vi "pp2_videoQueueMake.vi"(8 "error in":errorcluster, 11 "Camera":T3="cam0") -> (0 "error out":errorcluster, 1 "Image reference":T4, 2 "Session Out":T3, 3 "queue out":refnum<queue>)   [LabVIEW 2013]
uses:
  <vilib>/userdefined/High Color/IMAQdx.ctl
  <vilib>/vision/Image Controls.llb/IMAQ Image.ctl
  pp2_CTL_DaqConfig.ctl
  <vilib>/sound2/lvsound2.llb/Sound Output Task ID.ctl
  <vilib>/vision/driver/NI_Vision_Acquisition_Software.lvlib
panel:
  in  "Daq config 2":T1={"SW1 DI"="Dev1/port2/line0", "Code/Tone DO"="Dev1/port0:1", "Sound AO"="Dev2/ao0", "Shock intesity AO"="Dev1/ao1", "SW2 DI"="Dev1/port2/line1", "AO <=> Sound card"=FALSE, "sound card task"=0, "Variable shock"=FALSE, "Full code <=> Tone"=FALSE, "Webcam"="cam0", "Webcam on"=FALSE, "sound sample rate"=8000, "sound card\ndevice ID"=0} {"sound sample rate" min=8000; "sound card task" format="%.0x"}
  in  "Daq config":T1={"SW1 DI"="Dev1/port2/line0", "Code/Tone DO"="Dev1/port0:1", "Sound AO"="Dev2/ao0", "Shock intesity AO"="Dev1/ao1", "SW2 DI"="Dev1/port2/line1", "AO <=> Sound card"=FALSE, "sound card task"=0, "Variable shock"=FALSE, "Full code <=> Tone"=FALSE, "Webcam"="cam0", "Webcam on"=FALSE, "sound sample rate"=8000, "sound card\ndevice ID"=0} {"sound sample rate" min=8000; "sound card task" format="%.0x"}
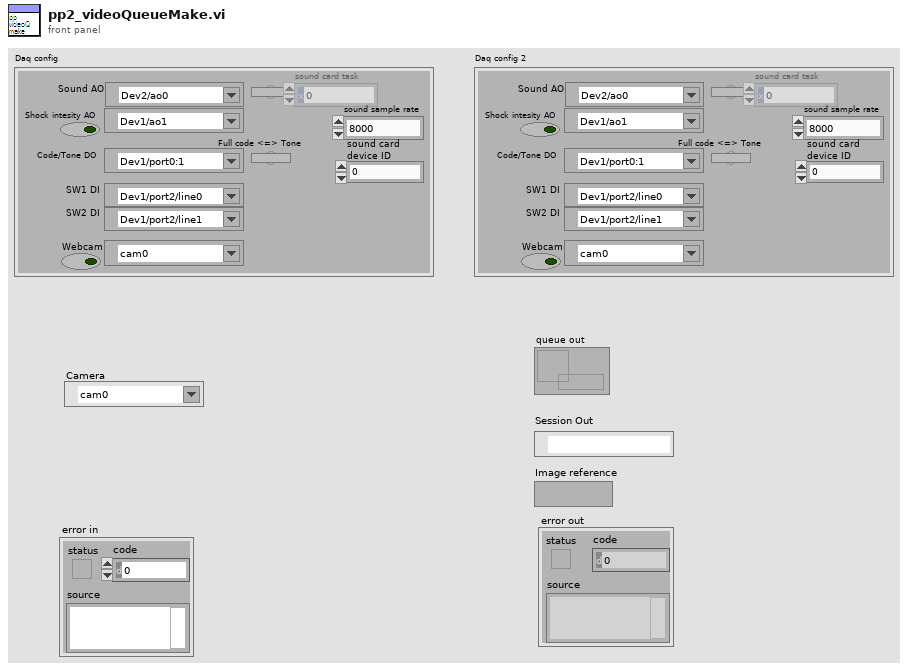
[diagram p1: front panel]
types:
  T1 = typedef "pp2_CTL_DaqConfig.ctl" = cluster{"SW1 DI":tag, "Code/Tone DO":tag, "Sound AO":tag, "Shock intesity AO":tag, "SW2 DI":tag, "AO <=> Sound card":bool, "sound card task":T2, "Variable shock":bool, "Full code <=> Tone":bool, "Webcam":T3, "Webcam on":bool, "sound sample rate":i32, "sound card\ndevice ID":u32}
  T2 = typedef "Sound Output Task ID.ctl" = u32
  T3 = typedef "IMAQdx.ctl" = refnum<k21>
  T4 = typedef "IMAQ Image.ctl" = refnum<image>
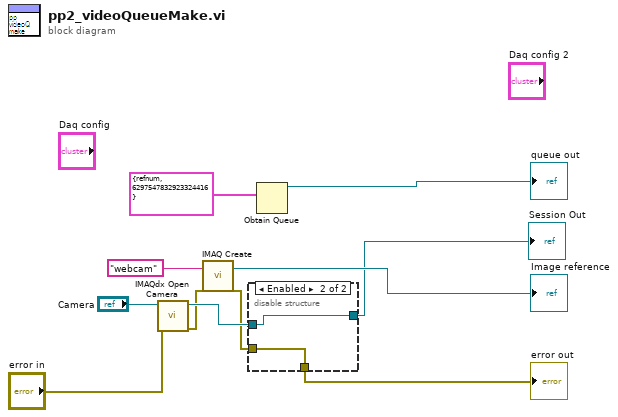
[diagram p0: block diagram]
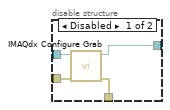
[diagram p2: hidden frame]
diagram:
  n1 = call <vilib>:"IMAQdx Open Camera.vi"("error in"="error in", "Session In"="Camera") -> ("error out"=w7:errorcluster, "Session Out"=w11:T3)  [unwired: 8 in]
  n2 = call "IMAQ Create"("Image Name"="webcam", "error in (no error)"=w7) -> ("New Image"=→"Image reference":T4, "error out"=w6:errorcluster)  [unwired: 3 in]
  n3 = disable-structure shown="Enabled" {
    disable-tunnel: w11 -> [w14 w17]
    disable-tunnel: w6 -> [w15 w16]
    disable-tunnel: [w13 w17] -> w2
    disable-tunnel: [w12 w16] -> w1
    frame Disabled {
      n4 = call <vilib>:"IMAQdx Configure Grab.vi"("error in"=w15, "Session In"=w14) -> ("error out"=w12:errorcluster, "Session Out"=w13:T3)  [unwired: 8 in]
    }
    frame Enabled {
    }
  }
  "Session Out" <- w2
  "error out" <- w1
  n5 = Obtain Queue(element data type=cluster{"Image":T4, i64} {"Image"="Webcam", 0}) -> (queue out=→"queue out":refnum<queue>)  [unwired: 4 in, 2 out]
